vi "UHR-Fleezers Control (host) - 10.8MV_trial2.vi"() -> ()   [LabVIEW 2010] (continued)
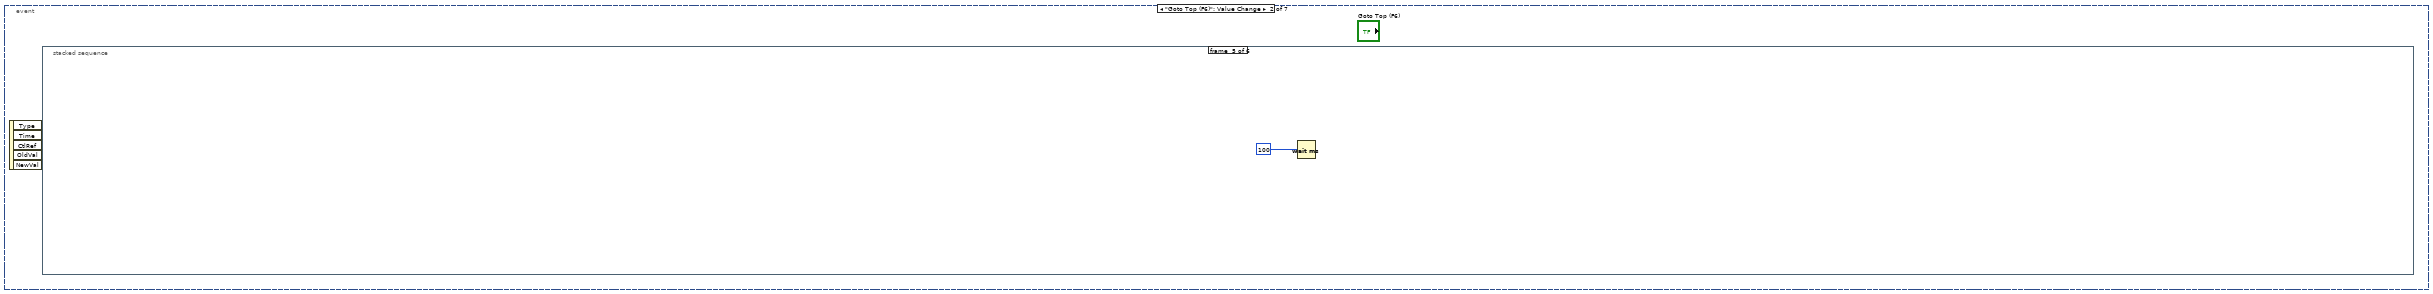
[diagram p3: hidden frame]
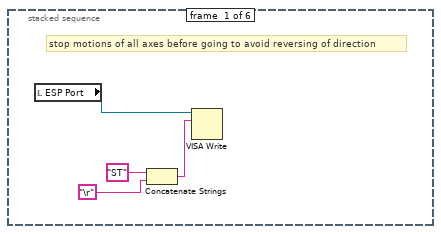
[diagram p4: hidden frame]
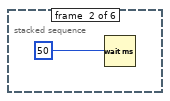
[diagram p5: hidden frame]
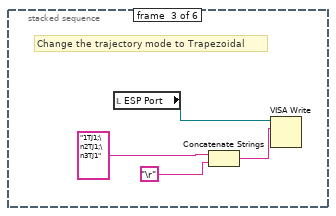
[diagram p6: hidden frame]
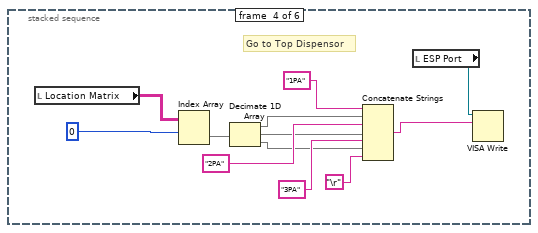
[diagram p7: hidden frame]
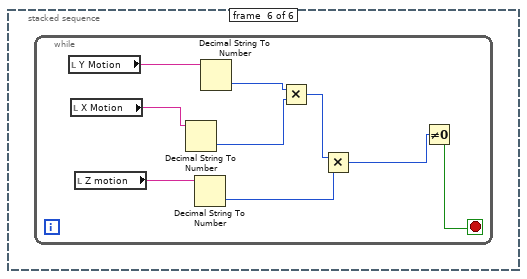
[diagram p8: hidden frame]
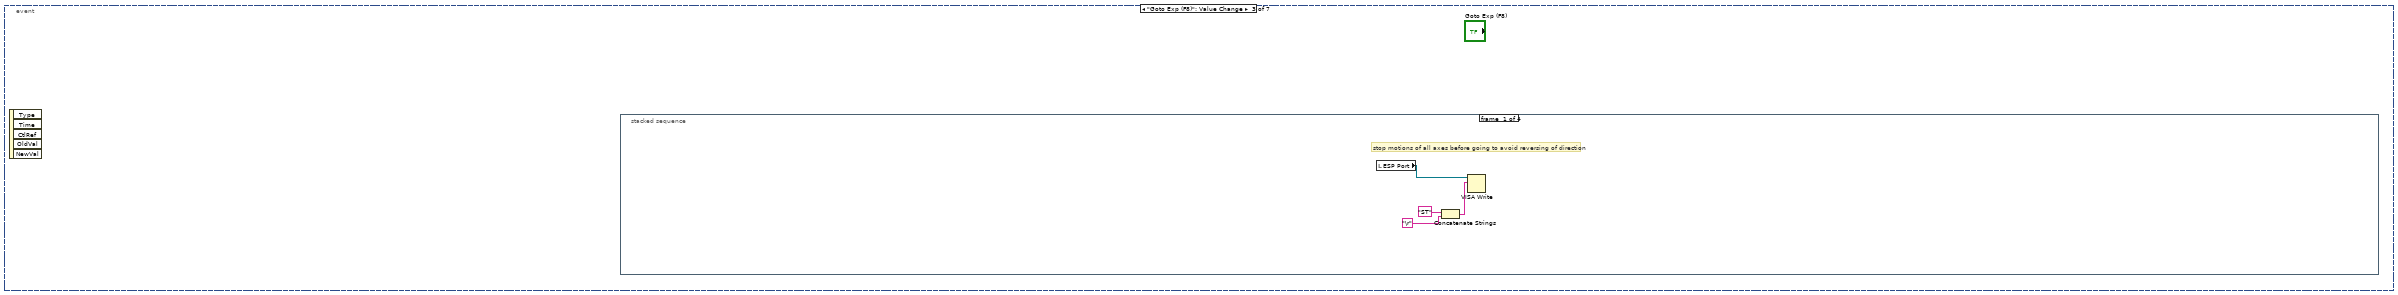
[diagram p9: hidden frame]
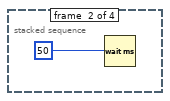
[diagram p10: hidden frame]
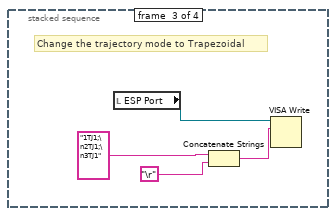
[diagram p11: hidden frame]
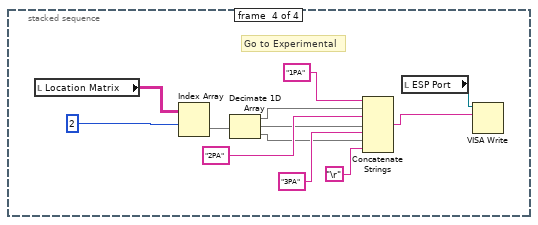
[diagram p12: hidden frame]
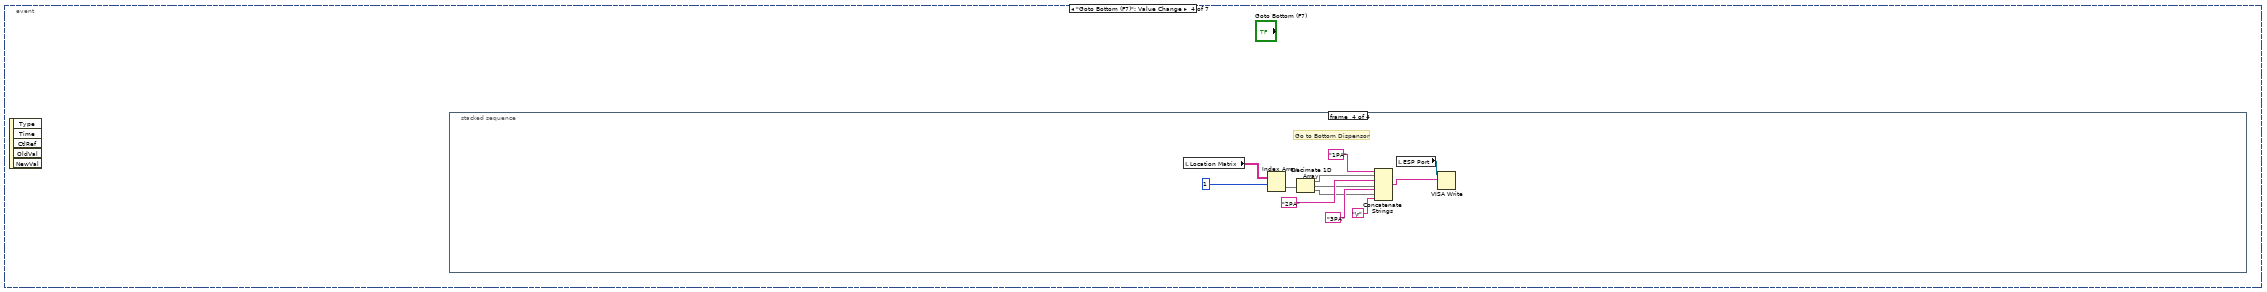
[diagram p13: hidden frame]
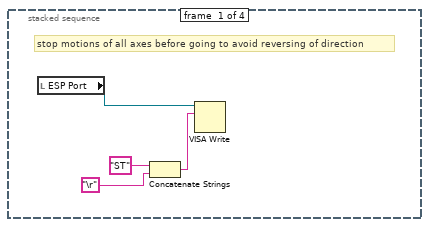
[diagram p14: hidden frame]
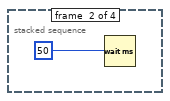
[diagram p15: hidden frame]
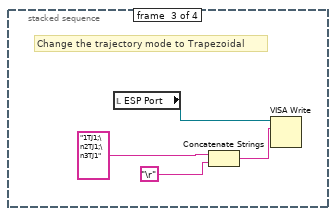
[diagram p16: hidden frame]
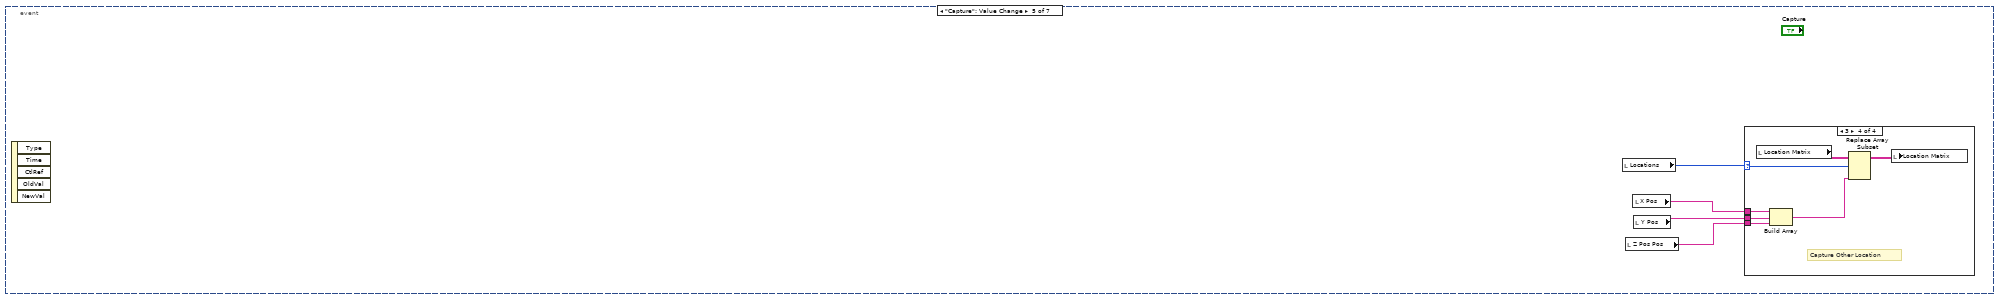
[diagram p17: hidden frame]
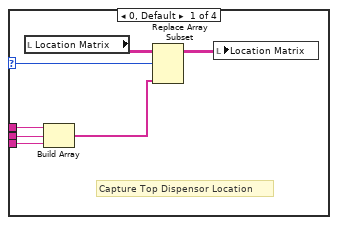
[diagram p18: hidden frame]
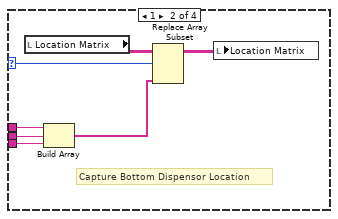
[diagram p19: hidden frame]
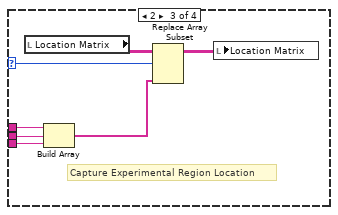
[diagram p20: hidden frame]
              tunnel: w8534 -> [_ w8614]
              tunnel: w8533 -> [_ w8568]
              tunnel: w8532 -> [_ w8607]
              tunnel: w8531 -> [_ w8585]
              tunnel: w8530 -> [w8553 w8566]
              tunnel: w8529 -> [w8554 w8565]
              tunnel: w8528 -> [_ w8562]
              frame False {
                w8552 = FALSE
                n1982 = Close File(refnum=w8558) -> ()  [unwired: 1 in, 2 out]
                n1983 = case shown="True" w8555 {
                  tunnel: w8556 -> [_ w8560]
                  frame False {
                  }
                  frame True {
                    n1984 = Close File(refnum=w8560) -> ()  [unwired: 1 in, 2 out]
                  }
                }
                n1985 = case shown="True" w8553 {
                  tunnel: w8554 -> [_ w8559]
                  frame False {
                  }
                  frame True {
                    n1986 = Close File(refnum=w8559) -> ()  [unwired: 1 in, 2 out]
                  }
                }
                n1987 = local write "Calibrating Trap..."(w8552) -> ()
                n1988 = call <vilib>:"Beep.vi"() -> ()  [unwired: 3 in, 9 out]
                n1989 = local write "Stop Saving"(w8552) -> ()
                n1990 = property on="Raster Scanning..." class="Bool (strict)"("Val(Sgnl)"=w8552) -> ()  [unwired: 2 in, 2 out]
                "Saving..." <- w8552
              }
              frame True {
                n1991 = local read "Calibrating Trap..."() -> (w8618:bool)
                n1992 = case "Write fl. data" shown="True" w8617 {
                  tunnel: w8616 -> [_ w8652]
                  tunnel: w8615 -> [_ w8651]
                  frame False {
                  }
                  frame True {
                    n1993 = Write to Binary File(file (use dialog)=w8652, data=w8651, 5:FALSE ("prepend array or string size? (T)"), 9:T31."big-endian, network order" ("byte order (0:big-endian, network order)")) -> ()  [unwired: 1 in, 4 out]
                  }
                }
                n1994 = Greater?(x="Save ave N", y=1.0) -> (0:w8621:bool)
                n1995 = Not(x=w8618) -> (.not. x?=w8620:bool)
                n1996 = And(x=w8620, y=w8621) -> (x .and. y?=w8563:bool)
                n1997 = case shown="True" w8563 {
                  tunnel: w8562 -> [w8632 w8643]
                  tunnel: [w8632 w8635] -> w8561
                  tunnel: "Save ave N" -> [_ w8636]
                  frame False {
                  }
                  frame True {
                    w8633 = 2 ("dimension size")
                    n1998 = Array Size(array=w8643) -> (size(s)=w8637:i32)
                    n1999 = Divide(x=w8637, y=w8633) -> (x/y=w8641:dbl)
                    n2000 = Reshape Array(w8643, w8641, w8633) -> (w8642:u64[][])
                    n2001 = Transpose 2D Array(2D array=w8642) -> (transposed array=w8640:u64[][])
                    n2002 = for {
                      tunnel: w8640 -> [w8645] mode=indexing
                      tunnel: [w8644] -> w8634 mode=indexing
                      tunnel: w8636 -> [w8646]
                      workers-P: _ -> [_]
                      n2003 = call "downsample 1D array - U64.vi"("Ave N"=w8646, "Array In"=w8645) -> ("Array Out"=w8644:u64[])  [unwired: 1 in]
                    }
                    n2004 = Transpose 2D Array(2D array=w8634) -> (transposed array=w8639:u64[][])
                    n2005 = Divide(x=w8637, y=w8636) -> (x/y=w8638:dbl)
                    n2006 = Reshape Array(w8639, w8638) -> (w8635:u64[])
                  }
                }
                n2007 = case shown="True" w8563 {
                  tunnel: w8623 -> [w8655 w8667]
                  tunnel: [w8655 w8659] -> w8619
                  tunnel: "Save ave N" -> [_ w8660]
                  tunnel: w8614 -> [_ w8658]
                  frame False {
                    # "don't downsample data for trap calibration"
                  }
                  frame True {
                    n2008 = Array Size(array=w8667) -> (size(s)=w8661:i32)
                    n2009 = Array Size(array=w8658) -> (size(s)=w8657:i32)
                    n2010 = Divide(x=w8661, y=w8657) -> (x/y=w8665:dbl)
                    n2011 = Reshape Array(w8667, w8665, w8657) -> (w8666:i16[][])
                    n2012 = Transpose 2D Array(2D array=w8666) -> (transposed array=w8664:i16[][])
                    n2013 = for {
                      tunnel: w8664 -> [w8670] mode=indexing
                      tunnel: [w8669] -> w8656 mode=indexing
                      tunnel: w8660 -> [w8668]
                      workers-P: _ -> [_]
                      n2014 = call "downsample 1D array - I16.vi"("Ave N"=w8668, "Array In"=w8670) -> ("Array Out"=w8669:i16[])  [unwired: 1 out]
                    }
                    n2015 = Transpose 2D Array(2D array=w8656) -> (transposed array=w8663:i16[][])
                    n2016 = Divide(x=w8661, y=w8660) -> (x/y=w8662:dbl)
                    n2017 = Reshape Array(w8663, w8662) -> (w8659:i16[])
                  }
                }
                n2018 = Index Array(array=w8585, index=1) -> (element=w8588:waveform(dbl))
                n2019 = Index Array(array=w8585, index=0) -> (element=w8590:waveform(dbl))
                n2020 = Unbundle By Name(w8588) -> ("Y"=w8592:dbl[])
                n2021 = Unbundle By Name(w8590) -> ("Y"=w8600:dbl[])
                n2022 = case "Write trap pos. data" shown="True" w8566 {
                  tunnel: w8565 -> [_ w8648]
                  tunnel: w8561 -> [_ w8647]
                  frame False {
                  }
                  frame True {
                    n2023 = Write to Binary File(file (use dialog)=w8648, data=w8647, 5:FALSE ("prepend array or string size? (T)"), 9:T31."big-endian, network order" ("byte order (0:big-endian, network order)")) -> ()  [unwired: 1 in, 4 out]
                  }
                }
                n2024 = Write to Binary File(file (use dialog)=w8626, data=w8619, 5:FALSE ("prepend array or string size? (T)"), 9:T31."big-endian, network order" ("byte order (0:big-endian, network order)")) -> ()  [unwired: 1 in, 4 out]
                n2025 = feedback #26(w8592) -> (w8594:dbl[])
                n2026 = Build Array (concatenate)(w8594, w8592) -> (w8593:dbl[])
                n2027 = Select(t=w8592, s=w8568, f=w8593) -> (s? t:f=w8578:dbl[])
                n2028 = feedback-in #26(w8578) -> ()
                n2029 = feedback #27(w8600) -> (w8613:dbl[])
                n2030 = Build Array (concatenate)(w8613, w8600) -> (w8612:dbl[])
                n2031 = Select(t=w8600, s=w8568, f=w8612) -> (s? t:f=w8587:dbl[])
                n2032 = feedback-in #27(w8587) -> ()
                n2033 = Divide(x=w8627, y=w8628) -> (x/y=w8630:dbl)
                n2034 = Multiply(x=w8630, y=100.0) -> (x*y=w8629:dbl)
                n2035 = Build Array(w8587, w8578) -> (→"Saved APD":dbl[][])
                n2036 = Array Size(array=w8587) -> (size(s)=w8605:i32)
                n2037 = Unbundle By Name(w8607) -> ("Y"=w8611:dbl[])
                n2038 = Subtract(x=w8605, y="N pts to average") -> (x-y=w8581:i32)
                n2039 = Multiply(x="N pts to average", y=u16 2) -> (x*y=w8582:u16)
                n2040 = Subtract(x=w8605, y=w8582) -> (x-y=w8580:i32)
                n2041 = feedback #28(w8611) -> (w8610:dbl[])
                n2042 = Build Array (concatenate)(w8610, w8611) -> (w8609:dbl[])
                n2043 = Select(t=w8611, s=w8568, f=w8609) -> (s? t:f=w8608:dbl[])
                "Trap Delta Graph" <- w8608
                n2044 = feedback-in #28(w8608) -> ()
                n2045 = Array Subset(array=w8587, index=w8581, length="N pts to average") -> (w8604:dbl[])
                n2046 = Array Subset(array=w8587, index=w8580, length="N pts to average") -> (w8603:dbl[])
                n2047 = Array Subset(array=w8578, index=w8581, length="N pts to average") -> (w8584:dbl[])
                n2048 = Array Subset(array=w8578, index=w8580, length="N pts to average") -> (w8583:dbl[])
                n2049 = call <vilib>:"Mean.vi"("X"=w8604) -> ("mean"=w8602:dbl)  [unwired: 1 out]
                n2050 = call <vilib>:"Mean.vi"("X"=w8584) -> ("mean"=w8577:dbl)  [unwired: 1 out]
                n2051 = call <vilib>:"Mean.vi"("X"=w8603) -> ("mean"=w8601:dbl)  [unwired: 1 out]
                n2052 = call <vilib>:"Mean.vi"("X"=w8583) -> ("mean"=w8576:dbl)  [unwired: 1 out]
                n2053 = Subtract(x=w8577, y=w8576) -> (x-y=w8567:dbl)
                "Delta Fl. 2" <- w8567
                n2054 = Subtract(x=w8602, y=w8601) -> (x-y=w8599:dbl)
                "Delta Fl. 1" <- w8599
                n2055 = Initialize Array(w8599, 1 ("dimension size")) -> (w8596:dbl[])
                n2056 = Initialize Array(w8567, 1 ("dimension size")) -> (w8573:dbl[])
                n2057 = feedback #29(w8596) -> (w8597:dbl[])
                n2058 = Build Array (concatenate)(w8597, w8596) -> (w8595:dbl[])
                n2059 = feedback #30(w8573) -> (w8574:dbl[])
                n2060 = Build Array (concatenate)(w8574, w8573) -> (w8572:dbl[])
                n2061 = Select(t=w8596, s=w8568, f=w8595) -> (s? t:f=w8571:dbl[])
                n2062 = feedback-in #29(w8571) -> ()
                n2063 = Select(t=w8573, s=w8568, f=w8572) -> (s? t:f=w8570:dbl[])
                n2064 = feedback-in #30(w8570) -> ()
                n2065 = Build Array(w8571, w8570) -> (→"Save APD Deriv":dbl[][])
              }
            }
            "Progress" <- w8544
            "Progress 2" <- w8544
          }
        }
      }
    }
    n2066 = Bundle By Name(cluster=w5587, "Green FB Ch 0"=w5586, "Green FB Ch 1"=w5585) -> (w5565:T50)
    "Green FB Signals (V)" <- w5565
    n2067 = Unbundle By Name(w5565) -> ("Green FB Ch 2"=→"Green FB Plot":dbl)
    n2068 = local read "wait to reset values"() -> (w5657:bool)
    n2069 = Not(x=w5654) -> (.not. x?=w5658:bool)
    n2070 = And(x=w5658, y=w5657) -> (x .and. y?=w5659:bool)
    n2071 = case "Part of MCL raster scanning: returns to initial positions after scan done" shown="True" w5659 {
      tunnel: w5662 -> [w7261 w7268]
      tunnel: [w7261 w7267] -> w5661
      tunnel: w5656 -> [w7260 w7266]
      tunnel: [w7260 w7265] -> w5655
      frame False {
      }
      frame True {
        w7276 = 10.0 ("y")
        w7275 = 32767.0 ("y")
        # "to return scan values\nafter a synchronous \nAOM scan"
        n2072 = local read "AO2"() -> (w7269:dbl)
        n2073 = local read "AO1"() -> (w7270:dbl)
        n2074 = local write "wait to reset values"(FALSE ("wait to reset values")) -> ()
        n2075 = Multiply(x=w7270, y=w7275) -> (x*y=w7272:dbl)
        n2076 = Multiply(x=w7269, y=w7275) -> (x*y=w7274:dbl)
        n2077 = Divide(x=w7272, y=w7276) -> (x/y=w7271:dbl)
        n2078 = Divide(x=w7274, y=w7276) -> (x/y=w7273:dbl)
        n2079 = To Word Integer(number=w7271) -> (16bit integer=w7277:i16)
        n2080 = To Word Integer(number=w7273) -> (16bit integer=w7278:i16)
        n2081 = local read "Total Counts (ticks)"() -> (w7262:u32)
        n2082 = xnode "Read/Write Control"("FPGA VI Reference In"=w7268, "error in"=w7266, "AO1"=w7277, "AO2"=w7278, "MCL count"=w7262) -> ("FPGA VI Reference Out"=w7267:T19, "error out"=w7265:errorcluster)
        n2083 = local read "Scan Range (V)\n(of steps)"() -> (w7263:dbl)
        n2084 = property on="Scan Range (V)\n(of steps)" class="DigNum (strict)"("Val(Sgnl)"=w7263) -> ()  [unwired: 2 in, 2 out]
      }
    }
    n2085 = node-c288() -> ()  [unwired: 2 out]
  }
  n2086 = node-c288(3 ("Processor")) -> (w74:T26)  [unwired: 3 out]
  n2087 = timed-loop "Oscillate AOD (debugging)" {
    tunnel: w24 -> [w8672]
    tunnel: [w8671] -> w36
    timing: w74 -> [_]
    timing-out: [_] -> w73
    stop <- w8671 stop-if-true
    n2088 = node-c288() -> ()  [unwired: 2 out]
    n2089 = event shown="[0] \"Oscillate Set 2\", \"Fish for Tether\": Value Change" {
      selector: _ -> [_ _ _]
      dyn-events: _ -> [_ _ _]
      timeout: _ -> [_ _ _]
      tunnel: w8672 -> [w8679 _ _]
      tunnel: [FALSE ("Stop All") _ w8947] -> w8671
      event "Oscillate Set 2", "Fish for Tether": Value Change {
        n2090 = event-data() -> ()  [unwired: 6 out]
        n2091 = local read "Oscillate Set 2"() -> (w8678:bool)
        n2092 = Or(x=w8678, y="Fish for Tether") -> (x .or. y?=w8676:bool)
        n2093 = case shown="True" w8676 {
          tunnel: w8679 -> [_ w8682]
          tunnel: "Fish for Tether" -> [_ w8681]
          frame False {
          }
          frame True {
            n2094 = case shown="True" w8681 {
              frame False {
              }
              frame True {
                n2095 = local write "Scan axis 2"(TRUE) -> ()
                n2096 = local write "Tether"(FALSE ("Tether")) -> ()
              }
            }
            n2097 = node-c288("Period") -> (w8684:T26)  [unwired: 3 out]
            n2098 = timed-loop "Oscillate AOD" {
              timing: w8684 -> [_]
              timing-out: [_] -> w8683
              tunnel: w8682 -> [w8694]
              tunnel: w8681 -> [w8693]
              i -> [w8696]
              stop <- w8692 stop-if-true
              n2099 = node-c288() -> (w8695:i64)  [unwired: 1 out]
              n2100 = flat-sequence {
                tunnel: w8696 -> [w8722]
                tunnel: w8695 -> [w8721]
                tunnel: w8694 -> [w8705]
                tunnel: w8693 -> [w8707]
                tunnel: [w8707] -> w8691
                tunnel: [w8706] -> w8690
                tunnel: [w8704] -> w8689
                tunnel: [w8701] -> w8687
                tunnel: w8691 -> [w8758]
                tunnel: w8690 -> [w8756]
                tunnel: w8689 -> [w8755]
                tunnel: [w8754] -> w8688
                tunnel: w8687 -> [w8753]
                tunnel: [w8822] -> w8692
                tunnel: w8688 -> [w8820]
                frame #0 {
                  n2101 = Divide(x=w8721, y=i64 1000) -> (x/y=w8716:dbl)
                  n2102 = Multiply(x=w8716, y=w8722) -> (x*y=w8718:dbl)
                  n2103 = Multiply(x="Osc. freq. (Hz)", y=6.283185307179586) -> (x*y=w8719:dbl)
                  n2104 = Multiply(x=w8719, y=w8718) -> (x*y=w8703:dbl)
                  n2105 = local read "BD 1 Frequency 2 (MHz)"() -> (w8700:dbl)
                  n2106 = local read "BD 1 Frequency 1 (MHz)"() -> (w8697:dbl)
                  n2107 = case shown="True" w8707 {
                    tunnel: w8703 -> [w8728 w8735]
                    tunnel: w8700 -> [_ w8745]
                    tunnel: [w8725 w8729] -> w8708
                    tunnel: [FALSE w8738] -> w8704
                    tunnel: [0.0 w8731] -> w8701
                    tunnel: w8697 -> [_ w8730]
                    frame False {
                      n2108 = Sine(x=w8728) -> (sin(x)=w8726:dbl)
                      n2109 = Multiply(x=w8726, y="Osc. amp. (MHz)") -> (x*y=w8725:dbl)
                    }
                    frame True {
                      n2110 = Cosine(x=w8735) -> (cos(x)=w8748:dbl)
                      n2111 = Subtract(x=w8745, y=w8730) -> (x-y=w8744:dbl)
                      n2112 = Decrement(x=w8748) -> (x-1=w8747:dbl)
                      n2113 = Subtract(x=w8744, y="Closest Delta (MHz)") -> (x-y=w8741:dbl)
                      n2114 = Divide(x=w8747, y=2.0) -> (x/y=w8742:dbl)
                      n2115 = Multiply(x=w8742, y=w8741) -> (x*y=w8729:dbl)
                      n2116 = local read "Vec Mean of T1 T2"() -> (w8737:dbl[])
                      n2117 = Greater?(x=w8737, y="Stop F (pN)") -> (0:w8739:bool[])
                      n2118 = Or Array Elements(Boolean array=w8739) -> (logical OR=w8738:bool)
                      n2119 = Divide(x=w8735, y=6.283185307179586) -> (x/y=w8734:dbl)
                      n2120 = Round Toward +Infinity(x=w8734) -> (ceil(x): smallest int >= x=w8731:dbl)
                      "Attempts" <- w8731
                      n2121 = Greater?(x=w8731, y="Attempt Limit") -> (0:w8733:bool)
                      n2122 = case shown="True" w8733 {
                        frame False {
                        }
                        frame True {
                          n2123 = local write "Fish for Tether"(FALSE ("Fish for Tether")) -> ()
                          n2124 = call <vilib>:"Beep.vi"() -> ()  [unwired: 3 in, 9 out]
                          n2125 = local read "Messages"() -> (w8750:string)
                          n2126 = call "Update messages.vi"("Message to add"="Tether fishing timeout." ("Messages"), "Old message string"=w8750) -> ("New message string"=→"Messages":string)
                        }
                      }
                    }
                  }
                  n2127 = local read "Y RF Frequency Limits (MHz)"() -> (w8709:T16)
                  n2128 = local read "X RF Frequency Limits (MHz)"() -> (w8710:T16)
                  n2129 = local read "BD 1 Frequency 3 (MHz)"() -> (w8715:dbl)
                  n2130 = local read "BD 2 Frequency 2 (MHz)"() -> (w8699:dbl)
                  n2131 = Select(t=w8700, s="Scan axis 2", f=w8699) -> (s? t:f=w8711:dbl)
                  n2132 = Add(x=w8708, y=w8711) -> (x+y=w8706:dbl)
                  n2133 = Select(t=w8706, s="Scan axis 2", f=w8700) -> (s? t:f=w8698:dbl)
                  n2134 = Select(t=w8699, s="Scan axis 2", f=w8706) -> (s? t:f=w8713:dbl)
                  n2135 = local read "BD 2 Frequency 3 (MHz)"() -> (w8714:dbl)
                  n2136 = call "set RF board frequency - interlace.vi"("Board 2 Frequency Limits"=w8709, "Board 1 Frequency Limits"=w8710, "FPGA VI Reference In"=w8705, "Board 2 Frequency 3 (MHz)"=w8714, "Board 1 Frequency 3 (MHz)"=w8715, "Board 2 Frequency 2 (MHz)"=w8699, "Board 2 Frequency 1 (MHz)"=w8713, "Board 1 Frequency 2 (MHz)"=w8698, "Board 1 Frequency 1  (MHz)"=w8697) -> ()  [unwired: 1 in, 2 out]
                }
                frame #1 {
                  n2137 = And(x=w8758, y=w8755) -> (x .and. y?=w8757:bool)
                  n2138 = case "Only if were fishing and now formed tether" shown="True" w8757 {
                    tunnel: w8756 -> [w8760 w8772]
                    tunnel: [w8759 w8771] -> w8754
                    tunnel: w8753 -> [_ w8767]
                    frame False {
                      n2139 = local read "Fish for Tether"() -> (w8759:bool)
                      n2140 = case shown="True" w8759 {
                        tunnel: w8760 -> [_ _]
                        frame False {
                        }
                        frame True {
                        }
                      }
                    }
                    frame True {
                      w8771 = FALSE ("Fish for Tether")
                      n2141 = call <vilib>:"Beep.vi"() -> ()  [unwired: 3 in, 9 out]
                      n2142 = Number To Decimal String(number=w8767, width (-)=i16 1) -> (decimal integer string=w8765:string)
                      n2143 = case shown="\"2\", \"3\", \"4\", \"5\", \"6\"" "Then..." {
                        selector: "Then..." -> [_ w8775]
                        tunnel: w8772 -> [w8774 _]
                        frame "1", Default {
                          # "do nothing"
                          n2144 = property on="BD 1 Frequency 1 (MHz)" class="DigNum (strict)"("Val(Sgnl)"=w8774) -> ()  [unwired: 2 in, 2 out]
                        }
                        frame "2", "3", "4", "5", "6" {
                          n2145 = flat-sequence {
                            tunnel: w8775 -> [w8777]
                            frame #0 {
                              n2146 = property on="Trap Delta (MHz)" class="DigNum (strict)"("Val(Sgnl)"="Move to Delta 1 (MHz)") -> ()  [unwired: 2 in, 2 out]
                            }
                            frame #1 {
                              n2147 = case shown="\"5\", \"6\"" w8777 {
                                selector: w8777 -> [w8780 w8790 _]
                                frame "3", "4" {
                                n2148 = flat-sequence {
                                tunnel: w8780 -> [w8781]
                                tunnel: [w8781] -> w8778
                                tunnel: [w8783] -> w8779
                                tunnel: w8778 -> [w8783]
                                tunnel: w8779 -> [w8787]
                                frame #0 {
                                n2149 = property on="Green Laser ON/Interlacing" class="Bool (strict)"("Val(Sgnl)"=TRUE ("Value (Signaling)")) -> ()  [unwired: 2 in, 2 out]
                                }
                                frame #1 {
                                n2150 = Multiply(x="Wait Before Save (s)", y=u32 1000 ("x")) -> (x*y=w8785:u32)
                                n2151 = Wait (ms)(milliseconds to wait=w8785) -> ()  [unwired: 1 out]
                                }
                                frame #2 {
                                n2152 = property on="Start Saving" class="Bool (strict)"("Value"=TRUE ("Start Saving")) -> ()  [unwired: 2 in, 2 out]
                                n2153 = case shown="Default" w8787 {
                                frame Default {
                                }
                                frame "4" {
                                n2154 = property on="Fl. Triggered..." class="Bool (strict)"("Val(Sgnl)"=TRUE ("Value (Signaling)")) -> ()  [unwired: 2 in, 2 out]
                                }
                                }
                                }
                                }
                                }
                                frame "5", "6" {
                                n2155 = stacked-sequence {
                                tunnel: w8790 -> [_ _ _ _ _ _ _ _ w8807 _ _]
                                frame #0 {
                                n2156 = Replace Array Subset(array=u32[] [0] ("Index Values"), new element="Raster Set Upon Tether", index=0) -> (w8791:u32[])
                                n2157 = property on="Saved AOD Raster Scan Parameter Sets" class="Arr (strict)"("Index Values"=w8791) -> ()  [unwired: 2 in, 2 out]
                                }
                                frame #1 {
                                n2158 = Wait (ms)(milliseconds to wait=u32 500) -> ()  [unwired: 1 out]
                                }
                                frame #2 {
                                n2159 = property on="Load parameters" class="Bool (strict)"("Val(Sgnl)"=TRUE ("Value (Signaling)")) -> ()  [unwired: 2 in, 2 out]
                                }
                                frame #3 {
                                n2160 = Wait (ms)(milliseconds to wait=u32 500) -> ()  [unwired: 1 out]
                                }
                                frame #4 {
                                n2161 = property on="Trap Raster Scan" class="Bool (strict)"("Val(Sgnl)"=TRUE ("Value (Signaling)")) -> ()  [unwired: 2 in, 2 out]
                                }
                                frame #5 {
                                n2162 = Wait (ms)(milliseconds to wait=u32 2000) -> ()  [unwired: 1 out]
                                }
                                frame #6 {
                                n2163 = while {
                                stop <- w8802 stop-if-true
                                n2164 = local read "Raster Scanning..."() -> (w8801:bool)
                                n2165 = local read "Saving..."() -> (w8804:bool)
                                n2166 = Wait (ms)(milliseconds to wait=u32 100) -> ()  [unwired: 1 out]
                                n2167 = Not(x=w8804) -> (.not. x?=w8803:bool)
                                n2168 = Not(x=w8801) -> (.not. x?=w8800:bool)
                                n2169 = And(x=w8803, y=w8800) -> (x .and. y?=w8802:bool)
                                }
                                }
                                frame #7 {
                                n2170 = property on="Trap Delta (MHz)" class="DigNum (strict)"("Val(Sgnl)"="Move to Delta 2 (MHz)") -> ()  [unwired: 2 in, 2 out]
                                }
                                frame #8 {
                                n2171 = local read "Tether"() -> (w8808:bool)
                                n2172 = case shown="True" w8808 {
                                tunnel: w8807 -> [_ w8809]
                                frame False {
                                }
                                frame True {
                                n2173 = flat-sequence {
                                tunnel: w8809 -> [w8811]
                                frame #0 {
                                n2174 = Wait (ms)(milliseconds to wait=u32 500) -> ()  [unwired: 1 out]
                                }
                                frame #1 {
                                n2175 = case shown="\"6\"" w8811 {
                                frame Default {
                                }
                                frame "6" {
                                n2176 = property on="Green Laser ON/Interlacing" class="Bool (strict)"("Val(Sgnl)"=TRUE ("Green Laser ON/Interlacing")) -> ()  [unwired: 2 in, 2 out]
                                }
                                }
                                }
                                frame #2 {
                                n2177 = Wait (ms)(milliseconds to wait=u32 500) -> ()  [unwired: 1 out]
                                }
                                frame #3 {
                                n2178 = local write "Start Saving"("Save at end (5, 6)") -> ()
                                }
                                }
                                }
                                }
                                }
                                frame #9 {
                                n2179 = local read "Bead Sep. Int. Time (s)"() -> (w8817:dbl)
                                n2180 = Multiply(x=w8817, y=1000.0) -> (x*y=w8816:dbl)
                                n2181 = Wait (ms)(milliseconds to wait=w8816) -> ()  [unwired: 1 out]
                                }
                                frame #10 {
                                n2182 = property on="Rescale on Mean" class="Bool (strict)"("Val(Sgnl)"=TRUE ("Value (Signaling)")) -> ()  [unwired: 2 in, 2 out]
                                }
                                }
                                }
                                frame "2", Default {
                                }
                              }
                            }
                          }
                        }
                      }
                      n2183 = Concatenate Strings("Formed tether in ", w8765, " attempt(s)." ("string")) -> (w8762:string)
                      n2184 = local read "Messages"() -> (w8769:string)
                      n2185 = local write "Fish for Tether"(w8771) -> ()
                      n2186 = call "Update messages.vi"("Message to add"=w8762, "Old message string"=w8769) -> ("New message string"=w8768:string)
                      n2187 = local write "Messages"(w8768) -> ()
                      n2188 = Get Date/Time In Seconds() -> (seconds since 1Jan1904=→"Time tether formed":timestamp)
                      "Tether" <- "Tether Alarm?"
                    }
                  }
                }
                frame #2 {
                  n2189 = local read "Oscillate Set 2"() -> (w8821:bool)
                  n2190 = local read "Stop All"() -> (w8823:bool)
                  n2191 = Not Or(1:w8820, 2:w8821) -> (0:w8819:bool)
                  n2192 = Compound Arithmetic op=OR(w8823, w8819) -> (w8822:bool)
                }
              }
              n2193 = node-c288() -> ()  [unwired: 2 out]
            }
            n2194 = node-c288(w8683) -> ()  [unwired: 1 out]
          }
        }
      }
      event "Fl. Triggered...": Value Change {
        n2195 = event-data() -> ()  [unwired: 7 out]
        n2196 = case shown="True" "Fl. Triggered..." {
          frame False {
          }
          frame True {
            n2197 = node-c288() -> (w8835:T26)  [unwired: 4 out]
            n2198 = timed-loop {
              timing: w8835 -> [_]
              timing-out: [_] -> w8834
              tunnel: "Action" -> [w8839]
              shift-right: [w8836] -> _
              shift-left: u8 255 -> [w8838]
              stop <- w8840 stop-if-true
              n2199 = node-c288() -> ()  [unwired: 2 out]
              n2200 = flat-sequence {
                tunnel: w8839 -> [w8852]
                tunnel: w8838 -> [w8849]
                tunnel: [w8848] -> w8837
                tunnel: [w8938] -> w8840
                tunnel: w8837 -> [w8937]
                tunnel: [w8937] -> w8836
                frame #0 {
                  n2201 = local read "Delta Fl. 2"() -> (w8843:dbl)
                  n2202 = local read "Delta Fl. 1"() -> (w8844:dbl)
                  n2203 = Select(t=w8844, s="APD to Watch", f=w8843) -> (s? t:f=w8842:dbl)
                  n2204 = Multiply(x="Fl. Delta Thresh. (kHz)", y=1000.0) -> (x*y=w8851:dbl)
                  n2205 = Greater?(x=w8842, y=w8851) -> (0:w8846:bool)
                  n2206 = Or(x="Force Yank", y=w8846) -> (x .or. y?=w8847:bool)
                  n2207 = case shown="True" w8847 {
                    tunnel: w8852 -> [_ w8862]
                    tunnel: w8849 -> [w8854 w8858]
                    tunnel: [w8854 w8855] -> w8848
                    frame False {
                    }
                    frame True {
                      n2208 = flat-sequence {
                        tunnel: w8859 -> [w8868]
                        tunnel: [w8868] -> w8863
                        tunnel: w8862 -> [w8867]
                        tunnel: [w8867] -> w8861
                        tunnel: [w8866] -> w8860
                        tunnel: w8858 -> [w8865]
                        tunnel: [w8864] -> w8857
                        tunnel: w8863 -> [w8893]
                        tunnel: w8861 -> [w8892]
                        tunnel: w8860 -> [w8891]
                        tunnel: w8857 -> [w8890]
                        tunnel: [w8890] -> w8856
                        tunnel: w8856 -> [w8935]
                        tunnel: [w8935] -> w8855
                        frame #0 {
                          n2209 = call <vilib>:"Beep.vi"() -> ()  [unwired: 3 in, 9 out]
                          n2210 = local write "Waiting"(FALSE ("Waiting")) -> ()
                          n2211 = Increment(x=w8865) -> (x+1=w8864:u8)
                          n2212 = case shown="\"Yank\"" w8867 {
                            tunnel: w8864 -> [_ _ w8874]
                            frame "Image" {
                              n2213 = property on="Confocal Image" class="Bool (strict)"("Val(Sgnl)"=TRUE ("Value (Signaling)")) -> ()  [unwired: 2 in, 2 out]
                            }
                            frame "Alarm", Default {
                            }
                            frame "Yank" {
                              n2214 = flat-sequence {
                                tunnel: w8874 -> [w8877]
                                tunnel: [w8876] -> w8873
                                tunnel: ["N Array El"] -> w8872
                                tunnel: w8873 -> [w8887]
                                tunnel: w8872 -> [w8883]
                                frame #0 {
                                n2215 = Multiply(x="Yank Delay (s)", y=1000.0) -> (x*y=w8880:dbl)
                                n2216 = Quotient & Remainder(x=w8877, y="N Array El") -> (x-y*floor(x/y)=w8876:u8)  [unwired: 1 out]
                                n2217 = Wait (ms)(milliseconds to wait=w8880) -> ()  [unwired: 1 out]
                                }
                                frame #1 {
                                n2218 = Random Number (0-1)() -> (number: 0 to 1=w8884:dbl)
                                n2219 = Multiply(x=w8883, y=w8884) -> (x*y=w8882:dbl)
                                n2220 = Round Toward -Infinity(1:w8882) -> (0:w8881:dbl)
                                n2221 = Select(t=w8881, s="Random Choice", f=w8887) -> (s? t:f=w8885:dbl)
                                n2222 = Index Array(array="Yank to Delta Array (MHz)", index=w8885) -> (element=w8888:dbl)
                                n2223 = property on="Trap Delta (MHz)" class="DigNum (strict)"("Val(Sgnl)"=w8888) -> ()  [unwired: 2 in, 2 out]
                                }
                              }
                            }
                          }
                          n2224 = local read "Time (s)"() -> (w8866:dbl)
                          "Fl. High" <- TRUE ("Yanking")
                        }
                        frame #1 {
                          n2225 = node-c288() -> (w8895:T26)  [unwired: 4 out]
                          n2226 = timed-loop {
                            timing: w8895 -> [_]
                            timing-out: [_] -> w8894
                            tunnel: w8893 -> [w8911]
                            tunnel: w8892 -> [w8909]
                            tunnel: w8891 -> [w8908]
                            stop <- w8910 stop-if-true
                            n2227 = node-c288() -> ()  [unwired: 2 out]
                            n2228 = local read "Fl. Delta Thresh. (kHz)"() -> (w8903:dbl)
                            n2229 = local read "Fl. Triggered..."() -> (w8912:bool)
                            n2230 = local read "Delta Fl. 1"() -> (w8899:dbl)
                            n2231 = local read "Delta Fl. 2"() -> (w8897:dbl)
                            n2232 = local read "Stop All"() -> (w8906:bool)
                            n2233 = local read "APD to Watch"() -> (w8898:bool)
                            n2234 = Select(t=w8899, s=w8898, f=w8897) -> (s? t:f=w8896:dbl)
                            n2235 = Not(x=w8912) -> (.not. x?=w8907:bool)
                            n2236 = Multiply(x=w8903, y=1000.0) -> (x*y=w8902:dbl)
                            n2237 = Negate(x=w8902) -> (-x=w8901:dbl)
                            n2238 = Less?(x=w8896, y=w8901) -> (x < y?=w8905:bool)
                            n2239 = Compound Arithmetic op=OR(w8905, w8906, w8907, "Force Reset") -> (w8910:bool)
                            n2240 = case shown="True" w8910 {
                              tunnel: w8911 -> [_ w8923]
                              tunnel: w8909 -> [_ w8922]
                              tunnel: w8908 -> [_ w8920]
                              frame False {
                              }
                              frame True {
                                n2241 = case shown="\"Yank\"" w8922 {
                                tunnel: w8923 -> [_ w8924]
                                frame "Image", Default {
                                }
                                frame "Yank" {
                                n2242 = flat-sequence {
                                tunnel: [w8929] -> w8925
                                tunnel: w8924 -> [w8929]
                                tunnel: w8925 -> [w8930]
                                frame #0 {
                                n2243 = local read "Yank Delay (s)"() -> (w8928:dbl)
                                n2244 = Multiply(x=w8928, y=1000.0) -> (x*y=w8926:dbl)
                                n2245 = Wait (ms)(milliseconds to wait=w8926) -> ()  [unwired: 1 out]
                                }
                                frame #1 {
                                n2246 = property on="Trap Delta (MHz)" class="DigNum (strict)"("Val(Sgnl)"=w8930) -> ()  [unwired: 2 in, 2 out]
                                }
                                }
                                }
                                }
                                n2247 = local read "Time (s)"() -> (w8921:dbl)
                                n2248 = Subtract(x=w8921, y=w8920) -> (x-y=w8917:dbl)
                                "Duration (s)" <- w8917
                                n2249 = Number To Decimal String(number=w8917, width (-)=i16 0) -> (decimal integer string=w8915:string)
                                n2250 = Concatenate Strings(w8915, " s fluorescence event." ("string")) -> (w8913:string)
                                n2251 = local read "Messages"() -> (w8919:string)
                                n2252 = call "Update messages.vi"("Message to add"=w8913, "Old message string"=w8919) -> ("New message string"=w8918:string)
                                n2253 = call <vilib>:"Beep.vi"() -> ()  [unwired: 3 in, 9 out]
                                n2254 = local write "Messages"(w8918) -> ()
                              }
                            }
                            n2255 = node-c288() -> ()  [unwired: 2 out]
                          }
                          n2256 = node-c288(w8894) -> ()  [unwired: 1 out]
                        }
                        frame #2 {
                          n2257 = local write "Fl. High"(FALSE ("Yanking")) -> ()
                        }
                      }
                      n2258 = local read "Trap Delta (MHz)"() -> (w8859:dbl)
                    }
                  }
                }
                frame #1 {
                  n2259 = local read "Stop All"() -> (w8941:bool)
                  n2260 = local read "Fl. Triggered..."() -> (w8939:bool)
                  n2261 = Not(x=w8939) -> (.not. x?=w8940:bool)
                  n2262 = Or(x=w8940, y=w8941) -> (x .or. y?=w8938:bool)
                  n2263 = Not(x=w8938) -> (.not. x?=→"Waiting":bool)
                }
              }
              n2264 = node-c288() -> ()  [unwired: 2 out]
            }
            n2265 = node-c288(w8834) -> ()  [unwired: 1 out]
          }
        }
      }
      event "Stop All": Value Change {
        n2266 = event-data() -> ()  [unwired: 7 out]
        n2267 = local read "Stop All"() -> (w8947:bool)
      }
    }
    n2268 = node-c288() -> ()  [unwired: 2 out]
  }
  n2269 = node-c288(w14) -> ()  [unwired: 1 out]
  n2270 = node-c288(w68) -> ()  [unwired: 1 out]
  n2271 = node-c288(w75) -> ()  [unwired: 1 out]
  n2272 = node-c288(w73) -> ()  [unwired: 1 out]
  n2273 = node-c288(w163) -> ()  [unwired: 1 out]
  n2274 = flat-sequence {
    tunnel: w33 -> [w8952]
    tunnel: [w8951] -> w39
    tunnel: [w8948] -> w38
    tunnel: w37 -> [_]
    tunnel: w36 -> [_]
    tunnel: w35 -> [_]
    tunnel: w34 -> [_]
    tunnel: w32 -> [w8949]
    tunnel: w39 -> [w9014]
    tunnel: w38 -> [w9013]
    frame #0 {
      w8950 = FALSE ("APD to FIFO")
      n2275 = xnode "Read/Write Control"("FPGA VI Reference In"=w8952, "error in"=w8949, "APD to FIFO"=w8950, "AI to FIFO"=w8950) -> ("FPGA VI Reference Out"=w8951:T19, "error out"=w8948:errorcluster)
    }
    frame #1 {
      n2276 = xnode "Invoke Method"("FPGA VI Reference In"=w9014, "error in"=w9013) -> ("FPGA VI Reference Out"=w9012:T19)  [unwired: 1 out]
      n2277 = xnode "Close FPGA VI Reference"("FPGA VI Reference In"=w9012) -> ()  [unwired: 1 in, 1 out]
    }
  }
